vi "Processor Open.vi"(0 "resource name":T2, 5 "bitfile path":path, 9 "force download":bool, 11 "error in":errorcluster) -> (4 "fpga reference out":T1, 15 "error out":errorcluster)   [LabVIEW 2019]
uses:
  <vilib>/userdefined/High Color/nirio_resource_hc.ctl
  TypeDefs/Blank FPGA Reference.ctl
  TypeDefs/Processor FPGA Reference.ctl
  <vilib>/FPGAPlugInAG/PXIe-7902R/niLvFpga_Open_PXIe-7902R.vi
  <vilib>/rvi/interface/common/dynamic/niFpgaDynamicAddResources.vi
  <vilib>/FPGAPlugInAG/Dynamic/niLvFpga_Download_Dynamic.vi
  <vilib>/FPGAPlugInAG/Dynamic/niLvFpga_Run_Dynamic.vi
  <vilib>/rvi/errors/niLvFpgaAdjustHostInterfaceError.vi
  <vilib>/rvi/interface/nirviOpenFPGA/nirviOpenFPGA.xnode
  FPGA Bitfiles/Processing Reference (3.072 GSps) 7902.lvbitx
  FPGA Bitfiles/Processing Reference (2.94912 GSps) 7902.lvbitx
  <vilib>/rvi/interface/nirviMethod/nirviMethod.xnode
  <vilib>/rvi/interface/nirviReadWriteControl/nirviReadWriteControl.xnode
  NiFpgaLv.dll
  <vilib>/rvi/interface/Simulation/niFpgaSimulationCallBeginRW.vi
panel:
  in  "timeout (s)":dbl=1.0 format="%#_13g"
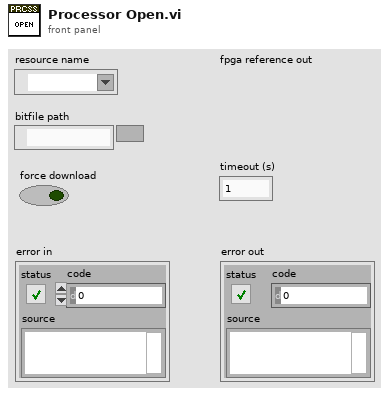
[diagram p1: front panel]
types:
  T1 = typedef "Blank FPGA Reference.ctl" = refnum<k20>
  T2 = typedef "nirio_resource_hc.ctl" = tag
  T3 = typedef "Processor FPGA Reference.ctl" = refnum<k20>
  T4 = typedef "Constants.ctl" = cluster{"data clock rate (Hz)":dbl, "sample rate (Hz)":dbl, "sample rate selector string":string, "default tx bitfile path":path, "default rx bitfile path":path, "default proc bitfile path":path}
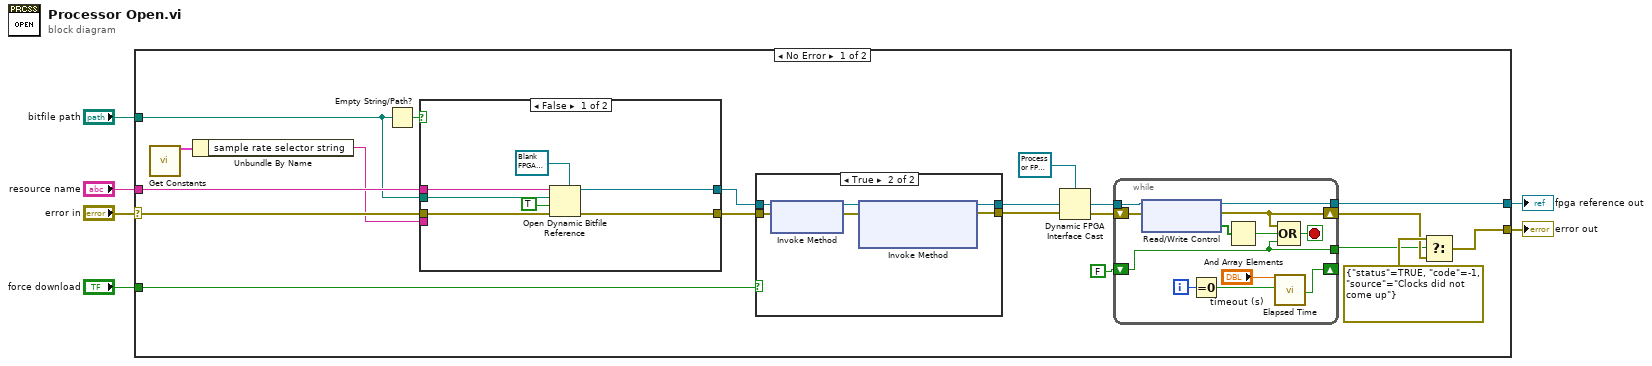
[diagram p0: block diagram]
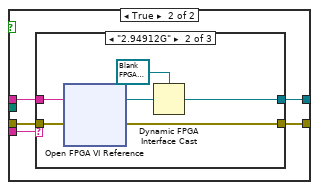
[diagram p2: hidden frame]
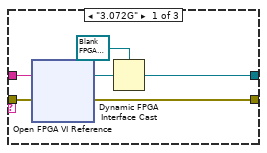
[diagram p3: hidden frame]
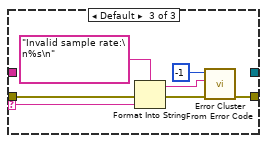
[diagram p4: hidden frame]
diagram:
  n1 = case shown="No Error" "error in" {
    selector: "error in" -> [w12 w77]
    tunnel: "resource name" -> [w10 _]
    tunnel: [w22 w77] -> w5
    tunnel: [w23 _] -> w2
    tunnel: "force download" -> [w25 _]
    tunnel: "bitfile path" -> [w8 _]
    frame No Error {
      n2 = call "Get Constants.vi"() -> ("constants"=w17:T4)  [unwired: 15 in]
      n3 = Unbundle By Name(w17) -> ("sample rate selector string"=w9:string)
      n4 = Empty String/Path?(string/path=w8) -> (empty?=w7:bool)
      n5 = case shown="False" w7 {
        tunnel: w12 -> [w28 w37]
        tunnel: w10 -> [w31 w36]
        tunnel: w9 -> [_ w35]
        tunnel: [w26 w34] -> w13
        tunnel: [w30 w33] -> w11
        tunnel: w8 -> [w27 _]
        frame False {
          n6 = Open Dynamic Bitfile Reference(0:w31, 1:w27, 2:TRUE ("Run When Loaded"), 3:w28, 4:T1 refnum ("blank fpga ref")) -> (5:w30:T1, 8:w26:errorcluster)
        }
        frame True {
          n7 = case shown="\"2.94912G\"" w35 {
            selector: w35 -> [_ _ w50]
            tunnel: w37 -> [w43 w49 w54]
            tunnel: w36 -> [w42 w48 _]
            tunnel: [w41 w47 w56] -> w34
            tunnel: [w38 w44 _] -> w33
            frame "3.072G" {
              n8 = xnode "Open FPGA VI Reference"("error in"=w43, "resource name"=w42) -> ("FPGA VI Reference Out"=w39:refnum<k20>, "error out"=w41:errorcluster)
              n9 = Dynamic FPGA Interface Cast(Session In=T1 refnum ("blank fpga ref"), Type=w39) -> (Session Out=w38:T1)
            }
            frame "2.94912G" {
              n10 = xnode "Open FPGA VI Reference"("error in"=w49, "resource name"=w48) -> ("FPGA VI Reference Out"=w46:refnum<k20>, "error out"=w47:errorcluster)
              n11 = Dynamic FPGA Interface Cast(Session In=T1 refnum ("blank fpga ref"), Type=w46) -> (Session Out=w44:T1)
            }
            frame Default {
              n12 = Format Into String(format string="Invalid sample rate:\n%s\n", error in=w54, w50) -> (resulting string=w52:string, error out=w53:errorcluster)  [unwired: 1 in]
              n13 = call <vilib>:"Error Cluster From Error Code.vi"("error in (no error)"=w53, "error message (\"\")"=w52, "error code (0)"=-1) -> ("error out"=w56:errorcluster)  [unwired: 6 in]
            }
          }
        }
      }
      n14 = case shown="True" w25 {
        tunnel: w11 -> [w70 w76]
        tunnel: [w69 w72] -> w24
        tunnel: w13 -> [w69 w74]
        tunnel: [w70 w71] -> w16
        frame False {
        }
        frame True {
          n15 = xnode "Invoke Method"("FPGA VI Reference In"=w76, "error in"=w74) -> ("FPGA VI Reference Out"=w75:T1, "error out"=w73:errorcluster)
          n16 = xnode "Invoke Method"("FPGA VI Reference In"=w75, "error in"=w73) -> ("FPGA VI Reference Out"=w71:T1, "error out"=w72:errorcluster)  [unwired: 1 in]
        }
      }
      n17 = Dynamic FPGA Interface Cast(Session In=T3 refnum ("FPGA VI Reference Out"), Type=w16) -> (Session Out=w15:T3)
      n18 = while {
        shift-right: [w66] -> w20
        shift-left: w24 -> [w68]
        tunnel: [w63] -> w19
        shift-right: [w59] -> _
        shift-left: FALSE ("Time has Elapsed") -> [w63]
        tunnel: w15 -> [w62]
        tunnel: [w61] -> w23
        i -> [w64]
        stop <- w65 stop-if-true
        n19 = xnode "Read/Write Control"("FPGA VI Reference In"=w62, "error in"=w68) -> ("FPGA VI Reference Out"=w61:T3, "error out"=w66:errorcluster, "clocks valid"=w60:bool[])
        n20 = Equal To 0?(x=w64) -> (x = 0?=w58:bool)
        n21 = And Array Elements(Boolean array=w60) -> (logical AND=w67:bool)
        n22 = call "Elapsed Time"("Time Target (s)"="timeout (s)", "Reset"=w58) -> ("Time has Elapsed"=w59:bool)  [unwired: 10 in, 7 out]
        n23 = Compound Arithmetic op=OR(w66, w67, w63) -> (w65:bool)
      }
      n24 = Select(t=errorcluster {"status"=TRUE, "code"=-1, "source"="Clocks did not come up"}, s=w19, f=w20) -> (s? t:f=w22:errorcluster)
    }
    frame Error {
    }
  }
  "error out" <- w5
  "fpga reference out" <- w2
